vi "CRYO_MASTER_temp_0911.vi"() -> ()   [LabVIEW 2017] (continued)
s since 1904-01-01), timestamp(3682565793.190962 s since 1904-01-01), timestamp(3682565794.192923 s since 1904-01-01), timestamp(3682565795.1943216 s since 1904-01-01), timestamp(3682565796.1945167 s since 1904-01-01), timestamp(3682565797.194023 s since 1904-01-01), timestamp(3682565798.195678 s since 1904-01-01), timestamp(3682565799.194545 s since 1904-01-01), timestamp(3682565800.194017 s since 1904-01-01), timestamp(3682565801.196416 s since 1904-01-01), timestamp(3682565802.1962314 s since 1904-01-01), timestamp(3682565803.1960993 s since 1904-01-01), timestamp(3682565804.196091 s since 1904-01-01), timestamp(3682565805.197301 s since 1904-01-01)], "DataArray"=[99.5330106117578]}] caption="XY Graph"
  in  "log/linear 4":bool
  in  "log/linear 3":bool
  in  "float/scientific 1":bool
  in  "P_safelimit_up (Pa)":dbl=300000.0 format="%_4e"
  in  "P_safelimit_low (Pa)":dbl=100.0 format="%_4e"
  out "Pav - (P_2_th_high+P_2_tol)=":dbl
  in  "Auto ON?":bool
  out "Pstd history":dbl(graph)=554.7391446242465
  out "Pav history":dbl(graph)=-49199.19854911039
  in  "Mov. Avg Interval":i64=4
  in  "V2 (N.C.)":bool
  in  "V1 (N.O.)":bool=TRUE
  in  "N for sampling":i64=7
  in  "P_2_tol (Pa)":dbl=5000.0 format="%_4e"
  in  "P_1_tol (Pa)":dbl=5000.0 format="%_4e"
  in  "P_2_th_low (Pa)":dbl=1.03 format="%_4e"
  in  "P_1_th_low (Pa)":dbl=125000.0 format="%_4g"
  in  "P_2_th_high (Pa)":dbl=1.2 format="%_4e"
  in  "P_1_th_high (Pa)":dbl=130000.0 format="%_4e"
  out "Graph 5":T9(graph) caption="XY Graph"
  out "Last N M.A. Pressures":dbl[](array[numeric]) format="%_5e"
  out "Pav":dbl=-49199.19854911039 format="%0.4e"
  out "Pstd":dbl=554.7391446242465 format="%0.4e"
  out "Status V2 CTRL":enum16{"Pressurize", "Depressurize"}(ring)
  out "Status V1 CTRL":enum16{"Pressurize", "Depressurize"}(ring)
  out "Pav - (P_2_th_low_-P_2_tol)=":dbl
  out "Pav - (P_1_th_low_-P_1_tol)=":dbl
  out "Pav - (P_1_th_high+P_1_tol)=":dbl
  out "File Refn DewarCTRL":refnum<file>
  out "Error Out (Dewar CTRL":errorcluster
  out "Actual Current (mA)":dbl min=0.0 max=1.9
  out "Graph 7":T10(graph) caption="XY Graph"
  in  "upper limit (V)":dbl=20.0 format="%#_13g"
  in  "lower limit (V)":dbl format="%#_13g"
  in  "lower limit (mA)":dbl=4.0
  in  "upper limit (mA) 2":dbl=20.0
  in  "lower limit (mA)":dbl=4.0
  in  "SetCurrent 2 (mA)":dbl
  in  "upper limit (mA)":dbl=20.0
  out "error out (KIKUSI CTRL)":errorcluster={"status"=TRUE, "code"=1, "source"="Format Into String in FileWrite.vi->CRYO_MASTER_temp.vi"}
  out "ActualVoltage (V)":dbl[](array[numeric])
  out "ActualCurrent (A)":dbl[](array[numeric])=[0.008, 0.01]
  in  "SetCurrent 1 (mA)":dbl
  in  "Output":bool[](array[boolean])=[FALSE, FALSE]
  out "error out (ADCMT6420A)":errorcluster
  in  "Voltage limits (V)":dbl[](array[numeric])=[12.0, 12.0]
  in  "CtrlLabels":string[](array[string])=["CV2", "CV3"]
  in  "VISA":refnum<visa-resource-name>[](array[refnum])=["GPIB0::1::INSTR", "GPIB0::12::INSTR"]
  out "Initialized?":bool
  in  "InstName":string="ADCMT"
  out "Graph 6":T9(graph) caption="XY Graph"
  in  "Initialize":bool
  in  "CONTROL KIKUSUI?":bool=TRUE
  in  "OUTPUT":bool
  in  "Set Voltage (V)":dbl=20.0 min=0.0 max=49.0
  in  "Set Current (mA)":dbl=0.001 min=0.0 max=1.9
  in  "offset (mA)":dbl=10.0 format="%#_13g"
  out "Series 1":string[](array[string])=["P_Dewar"]
  out "Series 2":string[](array[string])=["T4He6", "T4He9", "T3He1-2", "T3He1-3", "T4He7", "T4He8", "T4He10", "T1K6", "TIP1", "N.C.", "TIP2", "T1K3-1", "T1K3-2", "T3He5", "T3He8", "T3He6-1", "T3He6-2", "T3He7-1", "T3He7-2"]
  out "Series 3":string[](array[string])=["P_ins", "P_4Kres", "P_3HeIN", "P_SldRTN", "P_3Hepot", "P_1Kepot", "DP_HEX4", "DP_HEX5"]
  out "Series 4":string[](array[string])=["L1", "L2-1", "L2-2", "L3"]
  out "Plot errors":errorcluster
  out "LastMeasurementConfig (218)":T11(array[cluster])=[{"LSIName"="LSI218A", "Active?"=TRUE, "LastData"=[297.63, 297.76, 296.71, 297.24, 295.38, 295.52, 294.91, 295.07], "Labels"=["T3He10", "T3He1-1", "TTH3", "TTH4", "TTH1", "TTH2", "T4He1", "T1K1"]}, {"LSIName"="LSI218B", "Active?"=TRUE, "LastData"=[30.0, 0.0, 0.0, 0.0, 296.58, 296.99, 295.68, 297.19], "Labels"=["N.C.", "N.C.", "N.C.", "N.C.", "T3He2-1", "T3He2-2", "T3He3", "T3He1-4"]}, {"LSIName"="LSI218C", "Active?"=TRUE, "LastData"=[297.39, 297.55, 297.28, 297.31, 296.61, 296.28, 296.32, 296.17], "Labels"=["T4He3-1", "T4He3-2", "T4He3-3", "T4He3-4", "T4He2-1", "T4He2-2", "T4He4", "T4He5"]}, {"LSIName"="LSI218D", "Active?"=TRUE, "LastData"=[296.4, 297.17, 297.92, 297.51, 296.71, 297.02, 296.96, 297.42], "Labels"=["T4He6", "T4He9", "T3He1-2", "T3He1-3", "T4He7", "T4He8", "T4He10", "T1K6"]}, {"LSIName"="LSI218E", "Active?"=TRUE, "LastData"=[296.77, 0.0, 296.31, 688.49, 296.06, 295.63, 295.73, 688.58], "Labels"=["TIP1", "N.C.", "TIP2", "N.C.", "TIP3", "TIP4", "TIP5", "N.C."]}, {"LSIName"="LSI218F", "Active?"=TRUE, "LastData"=[302.11, 301.08, 296.91, 291.77, 288.69, 280.14, 0.433, 0.0], "Labels"=["T1K2", "T1K4", "T1K5", "T3He4", "T3He9", "TIP6", "N.C.", "N.C."]}]
  out "DataArrayConv (USB6210)":dbl[][](array[numeric])=[[0.000981756523507472, 101282.93029464335, 100447.56177003749, 100215.69769894995, 100421.61018172985, 100780.20754019849, 98878.77979362432, -9.626849444535207, 78.6252889928285, 100.08609659349952, 0.1296859810079549, 0.1356046075893618, 99.5330106117578]]
  out "LastMeasurementConfig (336)":T11(array[cluster])=[{"LSIName"="LSi336X", "Active?"=TRUE, "LastData"=[296.838, 296.434, 296.022, 296.217], "Labels"=["T1K3-1", "T1K3-2", "T3He5", "T3He8"]}, {"LSIName"="LSi336Y", "Active?"=TRUE, "LastData"=[295.887, 295.842, 295.916, 296.504], "Labels"=["T3He6-1", "T3He6-2", "T3He7-1", "T3He7-2"]}]
  out "DataArrayConv (USB6218)":dbl[][](array[numeric])
  out "TimeArray (USB6218)":timestamp[](array[timestamp])
  # "GLOBAL STATUS/CONTROL"
  # "USB6210 Analog inputs Settings"
  # "USB6218 Analog inputs Settings"
  # "USB6218 Digital Output Settings"
  # "USB6218 Analog Output Settings"
  # "Global Settings"
  # "LSI218 Settings"
  # "LSI336 Settings"
  # "Graph screenshots"
  # "Configuration"
  # "Vavle Status"
  # "OPEN"
  # "CLOSED"
  # "ADCMT6240A Control/Status"
  # "ADCMT6240A Initialization"
  # "Set Currents (mA)"
  # "KIKUSUI PWR400H CTRL via USB6218"
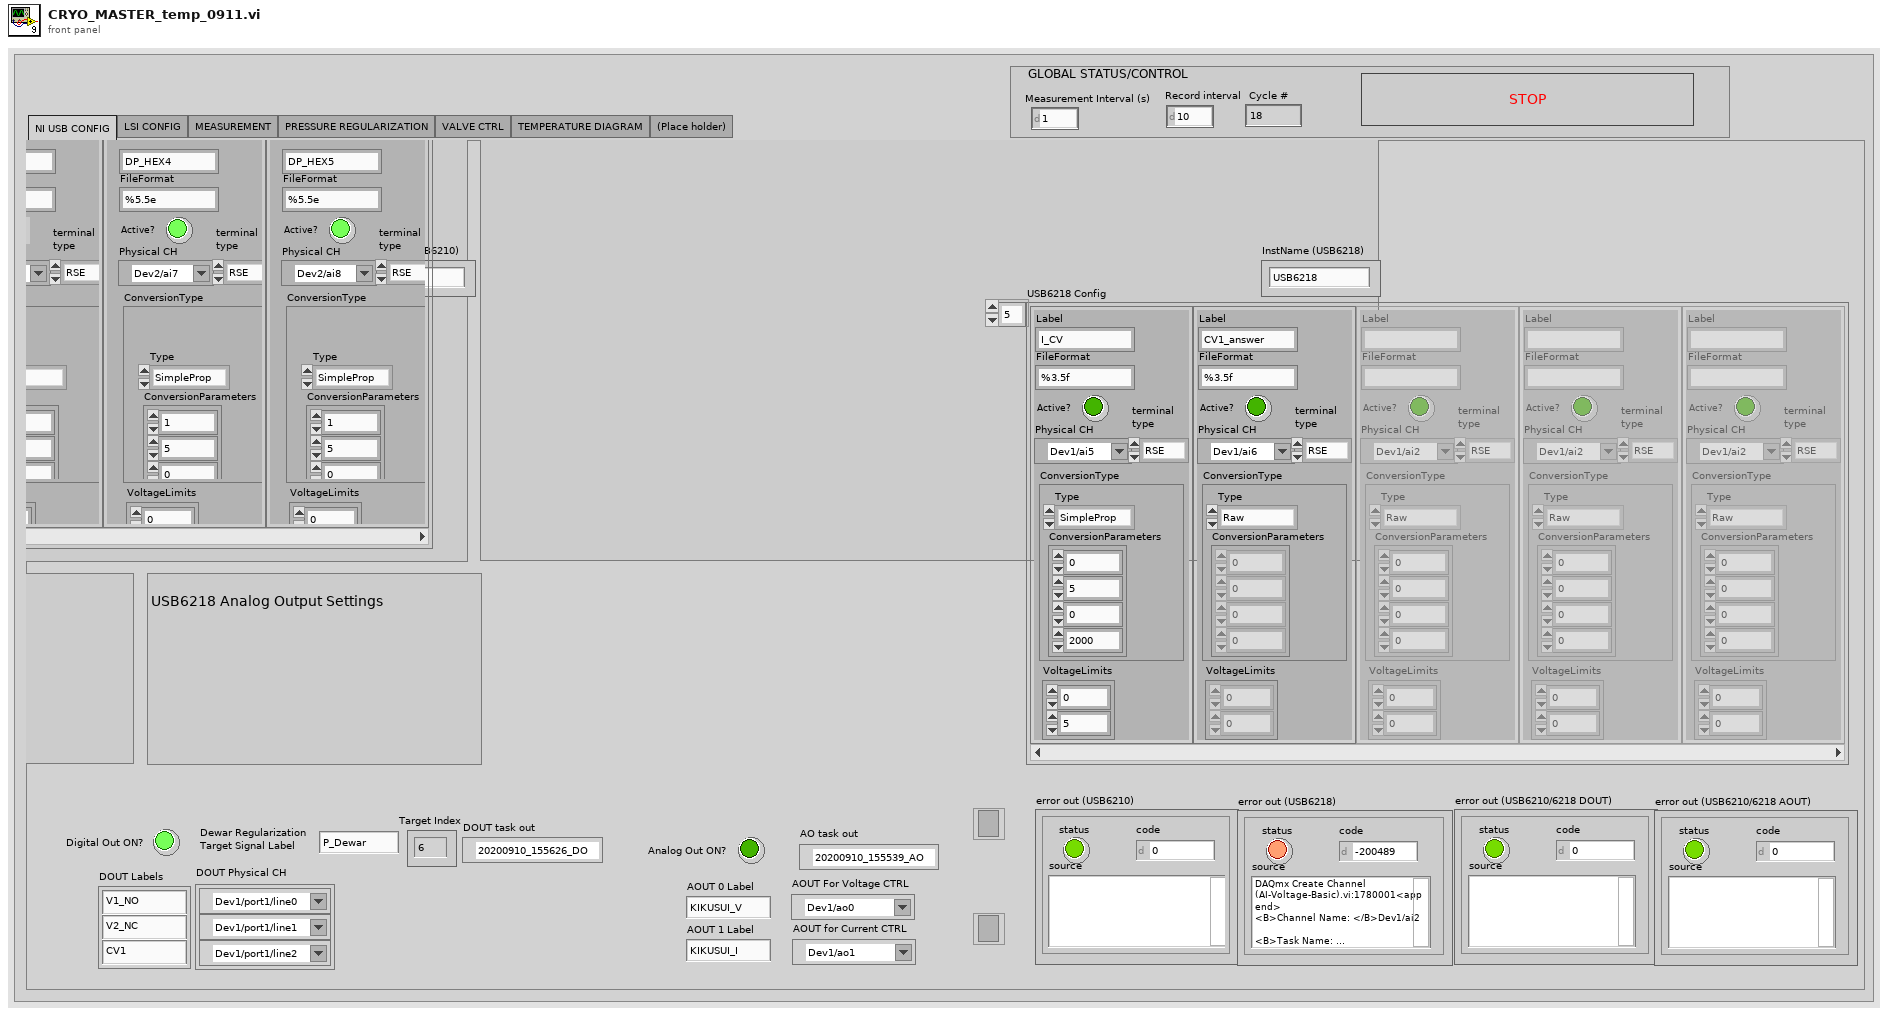
[diagram p1: front panel]
types:
  T1 = enum32{"NI USB CONFIG", "LSI CONFIG", "MEASUREMENT", "PRESSURE REGULARIZATION", "VALVE CTRL", "TEMPERATURE DIAGRAM", "(Place holder)"}
  T2 = cluster{"Label":string, "FileFormat":string, "Active?":bool, "Physical CH":tag, " terminal\n type":i32, "ConversionType":cluster{"Type":enum16{"Raw", "SimpleProp", "CC-10_COMBINED", "CC-10_LOG", "LeakDet_EXP", "LeakDet_Mantissa", "Baratron"}, "ConversionParameters":dbl[]}, "VoltageLimits":dbl[]}[]
  T3 = cluster{"LSIName":string, "Labels":string[], "SensorLocations":enum16{"N.C.", "T3He1-1", "T3He1-2", "T3He1-3", "T3He1-4", "T3He2-1", "T3He2-2", "T3He3", "T3He4", "T3He5", "T3He6-1", "T3He6-2", "T3He7-1", "T3He7-2", "T3He8", "T3He9", "T3He10", "T4He1", "T4He2-1", "T4He2-2", "T4He3-1", "T4He3-2", "T4He3-3", "T4He3-4", "T4He4", "T4He5", "T4He6", "T4He7", "T4He8", "T4He9", "T4He10", "T1K1", "T1K2", "T1K3-1", "T1K3-2", "T1K4", "T1K5", "T1K6", "TIP1", "TIP2", "TIP3", "TIP4", "TIP5", "TIP6", "TIP7", "TTH1", "TTH2", "TTH3", "TTH4"}[], "Active?":bool, "VISA res. name":refnum<visa-resource-name>}[]
  T4 = enum32{"USB6210", "USB6218", "Temeprature (1)", "Temperature (2)", "Temperature (3)"}
  T5 = enum16{"Intialized", "Ready", "Measuring", "Terminated"}
  T6 = enum16{"Initialized", "Ready", "Measuring", "Terminated"}
  T7 = cluster{"TimeArray":timestamp[], "LDArray":dbl[]}[]
  T8 = cluster{"TimeArray":timestamp[], "DataArray":dbl[]}[]
  T9 = cluster{"TimeArray":timestamp[], "Filtered X":dbl[]}[]
  T10 = cluster{"TimeArray (USB6218)":timestamp[], "DataArrayConv (USB6218)":dbl[]}[]
  T11 = cluster{"LSIName":string, "Active?":bool, "LastData":dbl[], "Labels":string[]}[]
  T12 = cluster{"TimeArray (USB6218)":timestamp[], "DataArrayConv (USB6218)":dbl[]}
  T13 = enum16{"open", "replace", "create", "open or create", "replace or create", "replace or create with confirmation"}
  T14 = cluster{"TimeArray":timestamp[], "DataArrayConv":dbl[]}[]
  T15 = cluster{"IndexArray":i64[], "TimeArray":timestamp[], "DataArrayRaw":dbl[][], "DataArrayConv":dbl[][], "LDArray":dbl[]}
  T16 = cluster{"InstName":string, "Active?":bool, "Status":enum16{"Intialized", "Ready", "Measuring", "Terminated"}, "Labels":string[], "LabelLD":string, "FileFormat":string[], "FileFormatLD":string, "ReadLeakDet?":bool}
  T17 = cluster{"TimeArray":timestamp[], "DataArrayConv":dbl[]}
  T18 = cluster{"TimeArray":timestamp[], "DataArray":dbl[]}
  T19 = cluster{"TimeArray":timestamp[], "Filtered X":dbl[]}
  T20 = cluster{"appended array":timestamp[], "ActualCurrentArray":dbl[]}
  T21 = cluster{"appended array":timestamp[], "SetCurrentArray":dbl[]}
  T22 = cluster{"appended array":timestamp[], "SetCurrentArray":dbl[]}[]
diagram:
  w3 = errorcluster {"status"=FALSE, "code"=0, "source"=""} ("error in (no error)")
  n1 = while {
    shift-right: [w38] -> _
    shift-left: dbl[] [] -> [w43]
    shift-right: [w39] -> _
    shift-left: timestamp[] [] -> [w42]
    i -> [w41]
    stop <- w51 stop-if-true
    n2 = stacked-sequence {
      tunnel: "upper limit (V)" -> [w58 w66 _]
      tunnel: "upper limit (mA) 2" -> [w56 w64 _]
      tunnel: "lower limit (V)" -> [w54 w62 _]
      tunnel: "Set Current (mA)" -> [w53 _ _]
      tunnel: [_ _ w73] -> w46
      tunnel: "Set Voltage (V)" -> [_ w61 _]
      tunnel: [_ _ w72] -> w44
      frame #0 {
        n3 = Greater?(x=w53, y=w58) -> (0:w57:bool)
        n4 = Less?(x=w53, y=w54) -> (x < y?=w55:bool)
        n5 = case shown="True" w57 {
          tunnel: w56 -> [_ w60]
          frame False {
          }
          frame True {
            n6 = property on="Set Current (mA)" class="DigNum (strict)"("Val(Sgnl)"=w60) -> ()  [unwired: 2 in, 2 out]
          }
        }
        n7 = case shown="True" w55 {
          tunnel: w54 -> [_ w59]
          frame False {
          }
          frame True {
            n8 = property on="Set Current (mA)" class="DigNum (strict)"("Val(Sgnl)"=w59) -> ()  [unwired: 2 in, 2 out]
          }
        }
      }
      frame #1 {
        n9 = Greater?(x=w61, y=w66) -> (0:w65:bool)
        n10 = Less?(x=w61, y=w62) -> (x < y?=w63:bool)
        n11 = case shown="True" w65 {
          tunnel: w64 -> [_ w68]
          frame False {
          }
          frame True {
            n12 = property on="Set Voltage (V)" class="DigNum (strict)"("Val(Sgnl)"=w68) -> ()  [unwired: 2 in, 2 out]
          }
        }
        n13 = case shown="True" w63 {
          tunnel: w62 -> [_ w67]
          frame False {
          }
          frame True {
            n14 = property on="Set Voltage (V)" class="DigNum (strict)"("Val(Sgnl)"=w67) -> ()  [unwired: 2 in, 2 out]
          }
        }
      }
      frame #2 {
        n15 = property on="Set Current (mA)" class="DigNum (strict)"() -> ("Value"=w71:dbl)  [unwired: 2 in, 2 out]
        n16 = Add(x=w71, y="offset (mA)") -> (x+y=w69:dbl)
        n17 = property on="Set Voltage (V)" class="DigNum (strict)"() -> ("Value"=w72:dbl)  [unwired: 2 in, 2 out]
        n18 = Divide(x=w69, y=1000.0) -> (x/y=w73:dbl)
      }
    }
    n19 = Wait (ms)(milliseconds to wait=u32 25) -> ()  [unwired: 1 out]
    n20 = event shown="[4] \"CONTROL KIKUSUI?\", \"Set Voltage (V)\", \"Set Current (mA)\": Value Change" {
      selector: _ -> [_ _ _ _ _ _]
      dyn-events: _ -> [_ _ _ _ _ _]
      timeout: _ -> [_ _ _ _ _ _]
      tunnel: [_ TRUE _ _ _ _] -> w51
      tunnel: w46 -> [_ _ _ _ w136 _]
      tunnel: w44 -> [_ _ _ _ w135 _]
      tunnel: w41 -> [_ _ _ _ w134 _]
      tunnel: [w76 w78 _ _ w133 w179] -> w38
      tunnel: w43 -> [w76 w78 _ _ w130 w179]
      tunnel: [w75 w77 _ _ w132 w180] -> w39
      tunnel: w42 -> [w75 w77 _ _ w131 w180]
      tunnel: w41 -> [_ _ w86 w107 _ w181]
      event Timeout {
        n21 = event-data() -> ()  [unwired: 1 in, 3 out]
      }
      event "Stop Button": Value Change {
        n22 = event-data() -> ()  [unwired: 1 in, 3 out]
        n23 = local read "AO task out"() -> (w80:refnum<k21>)
        n24 = local read "DOUT task out"() -> (w83:refnum<k21>)
        n25 = call <vilib>:"DAQmx Clear Task.vi"("task in"=w80, "error in"=errorcluster {"status"=FALSE, "code"=0, "source"=""}) -> ("error out"=w79:errorcluster)  [unwired: 13 in]
        n26 = call <vilib>:"DAQmx Clear Task.vi"("task in"=w83, "error in"=errorcluster {"status"=FALSE, "code"=0, "source"=""}) -> ("error out"=w84:errorcluster)  [unwired: 13 in]
        n27 = local write "error out (USB6210/6218 AOUT)"(w79) -> ()
        n28 = local write "error out (USB6210/6218 DOUT)"(w84) -> ()
      }
      event "V1 (N.O.)": Value Change {
        n29 = event-data() -> ()  [unwired: 1 in, 3 out]
        n30 = local read "Cycle #"() -> (w89:u32)
        n31 = Greater?(x=w89, y=u32 0) -> (0:w87:bool)
        n32 = case shown="True" w87 {
          tunnel: "V1 (N.O.)" -> [_ w99]
          tunnel: w86 -> [_ w94]
          frame False {
          }
          frame True {
            n33 = Not(x=w99) -> (.not. x?=w103:bool)
            n34 = local read "File Refn USB DO"() -> (w95:refnum<file>)
            n35 = local read "error out (USB6210/6218 DOUT)"() -> (w101:errorcluster)
            n36 = Initialize Array("%d" ("element"), 3 ("dimension size")) -> (w93:string[])
            n37 = property on="V2 (N.C.)" class="Bool (strict)"() -> ("Value"=w98:bool)  [unwired: 2 in, 2 out]
            n38 = property on="OUTPUT" class="Bool (strict)"() -> ("Value"=w97:bool)  [unwired: 2 in, 2 out]
            n39 = local read "DOUT task out"() -> (w106:refnum<k21>)
            n40 = Get Date/Time In Seconds() -> (seconds since 1Jan1904=w96:timestamp)
            n41 = call "FileWrite.vi"("Time Stamp"=w96, "FileFormat"=w93, "Index"=w94, "refnum in"=w95) -> ()  [unwired: 6 in, 2 out]
            n42 = Build Array(w103, w98, w97) -> (w102:bool[])
            n43 = call <vilib>:"DAQmx Write (Digital 1D Bool NChan 1Samp 1Line).vi"("task/channels in"=w106, "data"=w102, "timeout"=10.0, "error in"=w101) -> ("task out"=w104:refnum<k21>, "error out"=w100:errorcluster)  [unwired: 9 in, 1 out]
            n44 = local write "DOUT task out"(w104) -> ()
            n45 = local write "error out (USB6210/6218 DOUT)"(w100) -> ()
          }
        }
      }
      event "V2 (N.C.)": Value Change {
        n46 = event-data() -> ()  [unwired: 1 in, 3 out]
        n47 = local read "Cycle #"() -> (w110:u32)
        n48 = Greater?(x=w110, y=u32 0) -> (0:w108:bool)
        n49 = case shown="True" w108 {
          tunnel: "V2 (N.C.)" -> [_ w125]
          tunnel: w107 -> [_ w117]
          frame False {
          }
          frame True {
            n50 = property on="V1 (N.O.)" class="Bool (strict)"() -> ("Value"=w124:bool)  [unwired: 2 in, 2 out]
            n51 = local read "error out (USB6210/6218 DOUT)"() -> (w128:errorcluster)
            n52 = Not(x=w124) -> (.not. x?=w123:bool)
            n53 = property on="OUTPUT" class="Bool (strict)"() -> ("Value"=w122:bool)  [unwired: 2 in, 2 out]
            n54 = local read "DOUT task out"() -> (w129:refnum<k21>)
            n55 = Build Array(w123, w125, w122) -> (w120:bool[])
            n56 = local read "File Refn USB DO"() -> (w121:refnum<file>)
            n57 = Boolean To (0,1)(Boolean=w120) -> (0, 1=w119:i16[])
            n58 = call <vilib>:"DAQmx Write (Digital 1D Bool NChan 1Samp 1Line).vi"("task/channels in"=w129, "data"=w120, "timeout"=10.0, "error in"=w128) -> ("task out"=w126:refnum<k21>, "error out"=w113:errorcluster)  [unwired: 9 in, 1 out]
            n59 = Initialize Array("%d" ("element"), 3 ("dimension size")) -> (w114:string[])
            n60 = Get Date/Time In Seconds() -> (seconds since 1Jan1904=w118:timestamp)
            n61 = local write "DOUT task out"(w126) -> ()
            n62 = call "FileWrite.vi"("DataArray"=w119, "Time Stamp"=w118, "Error In"=w113, "FileFormat"=w114, "Index"=w117, "refnum in"=w121) -> ("Error Out"=w112:errorcluster)  [unwired: 4 in, 1 out]
            n63 = local write "error out (USB6210/6218 DOUT)"(w112) -> ()
          }
        }
      }
      event "CONTROL KIKUSUI?", "Set Voltage (V)", "Set Current (mA)": Value Change {
        n64 = event-data() -> ()  [unwired: 1 in, 3 out]
        n65 = case shown="True" "CONTROL KIKUSUI?" {
          tunnel: w136 -> [_ w153]
          tunnel: w135 -> [_ w158]
          tunnel: w134 -> [_ w161]
          tunnel: [w138 w151] -> w133
          tunnel: [w141 w150] -> w132
          tunnel: w131 -> [w143 w154]
          tunnel: w130 -> [w139 w152]
          frame False {
            w140 = 0.0 ("element")
            n66 = Get Date/Time In Seconds() -> (seconds since 1Jan1904=w142:timestamp)
            n67 = local read "AO task out"() -> (w148:refnum<k21>)
            n68 = Build Array (concatenate)(w143, w142) -> (w141:timestamp[])
            n69 = Build Array (concatenate)(w139, w140) -> (w138:dbl[])
            n70 = Build Array(w140, w140) -> (w146:dbl[])
            n71 = call <vilib>:"DAQmx Write (Analog 1D DBL NChan 1Samp).vi"("task/channels in"=w148, "data"=w146, "timeout"=100.0, "error in"=errorcluster {"status"=FALSE, "code"=0, "source"=""}) -> ("task out"=w149:refnum<k21>, "error out"=w144:errorcluster)  [unwired: 9 in, 1 out]
            n72 = local write "AO task out"(w149) -> ()
            n73 = local write "error out (KIKUSI CTRL)"(w144) -> ()
          }
          frame True {
            n74 = Build Array(w158, w153) -> (w156:dbl[])
            n75 = Divide(x=w153, y=2.0) -> (x/y=w171:dbl)
            n76 = Divide(x=w158, y=650.0) -> (x/y=w174:dbl)
            n77 = local read "File Refn USB AO"() -> (w162:refnum<file>)
            n78 = Multiply(x=10.0 ("y"), y=w174) -> (x*y=w169:dbl)
            n79 = Multiply(x=w171, y=10.0) -> (x*y=w168:dbl)
            n80 = Build Array(w169, w168) -> (w167:dbl[])
            n81 = Initialize Array("%.3f", 2 ("dimension size")) -> (w163:string[])
            n82 = Get Date/Time In Seconds() -> (seconds since 1Jan1904=w155:timestamp)
            n83 = local read "AO task out"() -> (w176:refnum<k21>)
            n84 = call "FileWrite.vi"("DataArray"=w156, "Time Stamp"=w155, "Error In"=errorcluster {"status"=FALSE, "code"=0, "source"=""} ("error in"), "FileFormat"=w163, "Index"=w161, "refnum in"=w162) -> ("Error Out"=w159:errorcluster, "Byte Stream File Refnum"=w157:refnum<file>)  [unwired: 4 in]
            n85 = Build Array (concatenate)(w154, w155) -> (w150:timestamp[])
            n86 = Build Array (concatenate)(w152, w153) -> (w151:dbl[])
            n87 = local write "File Refn USB AO"(w157) -> ()
            n88 = call <vilib>:"DAQmx Write (Analog 1D DBL NChan 1Samp).vi"("task/channels in"=w176, "data"=w167, "timeout"=100.0, "error in"=w159) -> ("task out"=w177:refnum<k21>, "error out"=→"error out (KIKUSI CTRL)":errorcluster)  [unwired: 9 in, 1 out]
            n89 = local write "AO task out"(w177) -> ()
          }
        }
      }
      event "OUTPUT": Value Change {
        n90 = event-data() -> ()  [unwired: 1 in, 6 out]
        n91 = local read "Cycle #"() -> (w184:u32)
        n92 = Greater?(x=w184, y=u32 0) -> (0:w182:bool)
        n93 = case shown="True" w182 {
          tunnel: w181 -> [_ w188]
          frame False {
          }
          frame True {
            n94 = property on="V1 (N.O.)" class="Bool (strict)"() -> ("Value"=w199:bool)  [unwired: 2 in, 2 out]
            n95 = local read "error out (USB6210/6218 DOUT)"() -> (w202:errorcluster)
            n96 = Not(x=w199) -> (.not. x?=w198:bool)
            n97 = property on="V2 (N.C.)" class="Bool (strict)"() -> ("Value"=w197:bool)  [unwired: 2 in, 2 out]
            n98 = local read "DOUT task out"() -> (w203:refnum<k21>)
            n99 = Build Array(w198, w197, "OUTPUT") -> (w186:bool[])
            n100 = Boolean To (0,1)(Boolean=w186) -> (0, 1=w185:i16[])
            n101 = local read "File Refn USB DO"() -> (w189:refnum<file>)
            n102 = call <vilib>:"DAQmx Write (Digital 1D Bool NChan 1Samp 1Line).vi"("task/channels in"=w203, "data"=w186, "timeout"=10.0, "error in"=w202) -> ("task out"=w200:refnum<k21>, "error out"=w193:errorcluster)  [unwired: 9 in, 1 out]
            n103 = Initialize Array("%d" ("element"), 3 ("dimension size")) -> (w191:string[])
            n104 = local write "DOUT task out"(w200) -> ()
            n105 = Get Date/Time In Seconds() -> (seconds since 1Jan1904=w190:timestamp)
            n106 = call "FileWrite.vi"("DataArray"=w185, "Time Stamp"=w190, "Error In"=w193, "FileFormat"=w191, "Index"=w188, "refnum in"=w189) -> ("Error Out"=w192:errorcluster, "Byte Stream File Refnum"=w187:refnum<file>)  [unwired: 4 in]
            n107 = local write "File Refn USB DO"(w187) -> ()
            n108 = local write "error out (USB6210/6218 DOUT)"(w192) -> ()
          }
        }
      }
    }
    n109 = local read "All Labels (USB6218)"() -> (w30:string[])
    n110 = Search 1D Array(1D array=w30, element="I_CV") -> (index of element=w28:i32)  [unwired: 1 in]
    n111 = local read "Last Data \n(USB6218)"() -> (w35:dbl[])
    n112 = Index Array(array=w35, index=w28) -> (element=→"Actual Current (mA)":dbl)
    n113 = local read "DataArrayConv (USB6218)"() -> (w31:dbl[][])
    n114 = Index Array(array=w31, index (row)=w28) -> (element=w32:dbl[])  [unwired: 1 in]
    n115 = local read "TimeArray (USB6218)"() -> (w33:timestamp[])
    n116 = Bundle(w39, w38) -> (w37:cluster{timestamp[], dbl[]})  [unwired: 1 in]
    n117 = Bundle("TimeArray (USB6218)"=w33, "DataArrayConv (USB6218)"=w32) -> (w36:T12)  [unwired: 1 in]
    n118 = Build Array(w37, w36) -> (→"Graph 7":T10)
  }
  n119 = while {
    stop <- w207 stop-if-true
    n120 = event shown="[5] \"float/scientific 1\": Value Change" {
      selector: _ -> [_ _ _ _ _ _ _ _ _ _ _ _]
      dyn-events: _ -> [_ _ _ _ _ _ _ _ _ _ _ _]
      timeout: _ -> [_ _ _ _ _ _ _ _ _ _ _ _]
      tunnel: [_ _ _ _ _ _ _ _ _ _ _ TRUE] -> w207
      event Timeout {
        n121 = event-data() -> ()  [unwired: 1 in, 3 out]
      }
      event "log/linear 1": Value Change {
        n122 = event-data() -> ()  [unwired: 1 in, 6 out]
        n123 = flat-sequence {
          frame #0 {
            n124 = control-ref of="Graph 1"() -> (w213:refnum<vi>)
            n125 = Boolean To (0,1)(Boolean="log/linear 1") -> (0, 1=w214:i16)
            n126 = property class="XYGraph (strict)"(reference=w213, error in=errorcluster {"status"=FALSE, "code"=0, "source"=""} ("error in (no error)"), "YScale.Mapping Mode"=w214) -> (error out=w211:errorcluster)  [unwired: 1 out]
            n127 = control-ref of="error out (USB6210)"() -> (w212:refnum<vi>)
            n128 = property class="Clust (strict)"(reference=w212, "Val(Sgnl)"=w211) -> ()  [unwired: 1 in, 2 out]
          }
        }
      }
      event "log/linear 2": Value Change {
        n129 = event-data() -> ()  [unwired: 1 in, 6 out]
        n130 = flat-sequence {
          frame #0 {
            n131 = control-ref of="Graph 2"() -> (w218:refnum<vi>)
            n132 = Boolean To (0,1)(Boolean="log/linear 2") -> (0, 1=w220:i16)
            n133 = property class="XYGraph (strict)"(reference=w218, error in=errorcluster {"status"=FALSE, "code"=0, "source"=""} ("error in (no error)"), "YScale.Mapping Mode"=w220) -> (error out=w219:errorcluster)  [unwired: 1 out]
            n134 = control-ref of="error out (USB6210)"() -> (w217:refnum<vi>)
            n135 = property class="Clust (strict)"(reference=w217, "Value"=w219) -> ()  [unwired: 1 in, 2 out]
          }
        }
      }
      event "log/linear 3": Value Change {
        n136 = event-data() -> ()  [unwired: 1 in, 6 out]
        n137 = flat-sequence {
          frame #0 {
            n138 = control-ref of="Graph 3"() -> (w222:refnum<vi>)
            n139 = Boolean To (0,1)(Boolean="log/linear 3") -> (0, 1=w226:i16)
            n140 = property class="XYGraph (strict)"(reference=w222, error in=errorcluster {"status"=FALSE, "code"=0, "source"=""} ("error in (no error)"), "YScale.Mapping Mode"=w226) -> (error out=w225:errorcluster)  [unwired: 1 out]
            n141 = control-ref of="error out (USB6210)"() -> (w224:refnum<vi>)
            n142 = property class="Clust (strict)"(reference=w224, "Value"=w225) -> ()  [unwired: 1 in, 2 out]
          }
        }
      }
      event "log/linear 4": Value Change {
        n143 = event-data() -> ()  [unwired: 1 in, 6 out]
        n144 = flat-sequence {
          frame #0 {
            n145 = control-ref of="Graph 4"() -> (w228:refnum<vi>)
            n146 = Boolean To (0,1)(Boolean="log/linear 4") -> (0, 1=w232:i16)
            n147 = property class="XYGraph (strict)"(reference=w228, error in=errorcluster {"status"=FALSE, "code"=0, "source"=""} ("error in (no error)"), "YScale.Mapping Mode"=w232) -> (error out=w231:errorcluster)  [unwired: 1 out]
            n148 = control-ref of="error out (USB6210)"() -> (w230:refnum<vi>)
            n149 = property class="Clust (strict)"(reference=w230, "Value"=w231) -> ()  [unwired: 1 in, 2 out]
          }
        }
      }
      event "float/scientific 1": Value Change {
        n150 = event-data() -> ()  [unwired: 1 in, 6 out]
        n151 = flat-sequence {
          frame #0 {
            n152 = control-ref of="Graph 4"() -> (w236:refnum<vi>)
            n153 = case shown="False" "float/scientific 1" {
              tunnel: [u8 1 ("Y Scale.Display Format:Format") u8 2 ("Y Scale.Display Format:Format")] -> w235
              frame False {
              }
              frame True {
              }
            }
            n154 = property class="XYGraph (strict)"(reference=w236, error in=errorcluster {"status"=FALSE, "code"=0, "source"=""} ("error in (no error)"), "YScale.Format"=w235) -> (error out=w238:errorcluster)  [unwired: 1 out]
            n155 = control-ref of="error out (USB6210)"() -> (w237:refnum<vi>)
            n156 = property class="Clust (strict)"(reference=w237, "Value"=w238) -> ()  [unwired: 1 in, 2 out]
          }
        }
      }
      event "Plot selecter LSI218(1)\n    1      2     3     4", "Plot selecter LSI218(2)\n    1      2     3     4", "Plot selecter (USB6210)\n    1      2     3     4", "Plot selecter LSI336 \n     1      2     3     4", "Plot selecter (USB6218)\n    1      2     3     4": Value Change {
        n157 = event-data() -> ()  [unwired: 1 in, 6 out]
        n158 = local read "All Labels (USB6210)"() -> (w258:string[])
        n159 = local read "All Labels (USB6218)"() -> (w247:string[])
        n160 = local read "Labels LSI218 (1)"() -> (w260:string[])
        n161 = local read "Labels LSI218 (2)"() -> (w261:string[])
        n162 = local read "Labels LSI336"() -> (w253:string[])
        n163 = call "BuildPlotLegends.vi"("Plot selecter \n    1      2     3     4"="Plot selecter (USB6210)\n    1      2     3     4", "AllLabels"=w258) -> ("Series 4"=w270:string[], "Series 3"=w268:string[], "Series 2"=w266:string[], "Series 1"=w264:string[])  [unwired: 6 in]
        n164 = call "BuildPlotLegends_LSI218.vi"("Plot selecter (2)\n    1      2     3     5"="Plot selecter LSI218(2)\n    1      2     3     4", "Plot selecter (1)\n    1      2     3     4"="Plot selecter LSI218(1)\n    1      2     3     4", "Labels (2)"=w261, "Labels (1)"=w260) -> ("Series 4"=w271:string[], "Series 3"=w269:string[], "Series 2"=w267:string[], "Series 1"=w265:string[])  [unwired: 4 in]
        n165 = call "BuildPlotLegends.vi"("Plot selecter \n    1      2     3     4"="Plot selecter LSI336 \n     1      2     3     4", "AllLabels"=w253) -> ("Series 4"=w248:string[], "Series 3"=w249:string[], "Series 2"=w250:string[], "Series 1"=w251:string[])  [unwired: 6 in]
        n166 = call "BuildPlotLegends.vi"("Plot selecter \n    1      2     3     4"="Plot selecter (USB6218)\n    1      2     3     4", "AllLabels"=w247) -> ("Series 4"=w243:string[], "Series 3"=w242:string[], "Series 2"=w244:string[], "Series 1"=w245:string[])  [unwired: 6 in]
        n167 = Build Array (concatenate)(w266, w267, w250, w244) -> (w255:string[])
        "Series 2" <- w255
        n168 = Build Array (concatenate)(w268, w269, w249, w242) -> (w256:string[])
        "Series 3" <- w256
        n169 = Build Array (concatenate)(w270, w271, w248, w243) -> (w257:string[])
        "Series 4" <- w257
        n170 = Build Array (concatenate)(w264, w265, w251, w245) -> (w254:string[])
        "Series 1" <- w254
        n171 = stacked-sequence {
          tunnel: [w280 _ _ _] -> w275
          tunnel: [_ w299 _ _] -> w276
          tunnel: [_ _ w315 _] -> w274
          tunnel: [_ _ _ w332] -> w273
          tunnel: w254 -> [w277 _ _ _]
          tunnel: w255 -> [_ w295 _ _]
          tunnel: w256 -> [_ _ w312 _]
          tunnel: w257 -> [_ _ _ w329]
          frame #0 {
            n172 = Array Size(array=w277) -> (size(s)=w283:i32)
            n173 = control-ref of="Graph 1"() -> (w281:refnum<vi>)
            n174 = for {
              N: 18 -> [_]
              tunnel: w281 -> [w292]
              shift-right: [w290] -> w282
              shift-left: errorcluster {"status"=FALSE, "code"=0, "source"=""} ("error in (no error)") -> [w291]
              i -> [w294]
              n175 = property class="XYGraph (strict)"(reference=w292, error in=w291, "Active Plot"=w294, "Plot.Plot Name"="") -> (error out=w290:errorcluster)  [unwired: 1 out]
            }
            n176 = for {
              N: w283 -> [_]
              tunnel: w281 -> [w288]
              shift-right: [w286] -> w280
              shift-left: w282 -> [w287]
              tunnel: w277 -> [w285] mode=indexing
              i -> [w289]
              n177 = property class="XYGraph (strict)"(reference=w288, error in=w287, "Active Plot"=w289, "Plot.Plot Name"=w285, "Plot.Visible?"=TRUE ("Plot.Visible")) -> (error out=w286:errorcluster)  [unwired: 1 out]
            }
          }
          frame #1 {
            n178 = Array Size(array=w295) -> (size(s)=w301:i32)
            n179 = control-ref of="Graph 2"() -> (w298:refnum<vi>)
            n180 = for {
              N: 18 -> [_]
              shift-right: [w308] -> w300
              shift-left: errorcluster {"status"=FALSE, "code"=0, "source"=""} ("error in (no error)") -> [w309]
              tunnel: w298 -> [w307]
              i -> [w311]
              n181 = property class="XYGraph (strict)"(reference=w307, error in=w309, "Active Plot"=w311, "Plot.Plot Name"="") -> (error out=w308:errorcluster)  [unwired: 1 out]
            }
            n182 = for {
              N: w301 -> [_]
              shift-right: [w304] -> w299
              shift-left: w300 -> [w305]
              tunnel: w295 -> [w303] mode=indexing
              tunnel: w298 -> [w302]
              i -> [w306]
              n183 = property class="XYGraph (strict)"(reference=w302, error in=w305, "Active Plot"=w306, "Plot.Plot Name"=w303) -> (error out=w304:errorcluster)  [unwired: 1 out]
            }
          }
          frame #2 {
            n184 = Array Size(array=w312) -> (size(s)=w318:i32)
            n185 = control-ref of="Graph 3"() -> (w316:refnum<vi>)
            n186 = for {
              N: 18 -> [_]
              tunnel: w316 -> [w326]
              shift-right: [w324] -> w317
              shift-left: errorcluster {"status"=FALSE, "code"=0, "source"=""} ("error in (no error)") -> [w325]
              i -> [w328]
              n187 = property class="XYGraph (strict)"(reference=w326, error in=w325, "Active Plot"=w328, "Plot.Plot Name"="") -> (error out=w324:errorcluster)  [unwired: 1 out]
            }
            n188 = for {
              N: w318 -> [_]
              tunnel: w316 -> [w322]
              shift-right: [w320] -> w315
              shift-left: w317 -> [w321]
              tunnel: w312 -> [w319] mode=indexing
              i -> [w323]
              n189 = property class="XYGraph (strict)"(reference=w322, error in=w321, "Active Plot"=w323, "Plot.Plot Name"=w319) -> (error out=w320:errorcluster)  [unwired: 1 out]
            }
          }
          frame #3 {
            n190 = Array Size(array=w329) -> (size(s)=w335:i32)
            n191 = control-ref of="Graph 4"() -> (w333:refnum<vi>)
            n192 = for {
              N: 18 -> [_]
              tunnel: w333 -> [w343]
              shift-right: [w341] -> w334
              shift-left: errorcluster {"status"=FALSE, "code"=0, "source"=""} ("error in (no error)") -> [w342]
              i -> [w345]
              n193 = property class="XYGraph (strict)"(reference=w343, error in=w342, "Active Plot"=w345, "Plot.Plot Name"="") -> (error out=w341:errorcluster)  [unwired: 1 out]
            }
            n194 = for {
              N: w335 -> [_]
              tunnel: w333 -> [w339]
              shift-right: [w337] -> w332
              shift-left: w334 -> [w338]
              tunnel: w329 -> [w336] mode=indexing
              i -> [w340]
              n195 = property class="XYGraph (strict)"(reference=w339, error in=w338, "Active Plot"=w340, "Plot.Plot Name"=w336) -> (error out=w337:errorcluster)  [unwired: 1 out]
            }
          }
        }
        n196 = Merge Errors(w275, w276, w274, w273) -> (→"Plot errors":errorcluster)
      }
      event "Take Screenshot! 1": Value Change {
        n197 = event-data() -> ()  [unwired: 1 in, 6 out]
        n198 = flat-sequence {
          frame #0 {
            n199 = flat-sequence {
              frame #0 {
                w349 = "_" ("string")
                n200 = Get Date/Time In Seconds() -> (seconds since 1Jan1904=w346:timestamp)
                n201 = local read "RUN identifier"() -> (w353:string)
                n202 = call "LV_UNIXTIME.vi"("current time"=w346) -> ("date/time string"=w350:string)  [unwired: 9 in, 1 out]
                n203 = local read "Base Path"() -> (w354:path)
                n204 = Concatenate Strings(w353, w349, w350, w349, "FIle suffix 1", ".bmp" ("string")) -> (w359:string)
                n205 = control-ref of="Graph 1"() -> (w351:refnum<vi>)
                n206 = Build Path(base path=w354, name or relative path=w359) -> (appended path=w358:path)
                n207 = invoke on="Invoke Node" class="XYGraph (strict)" method="Export Image"(reference=w351, "FileType"=enum32{"BMP", "EPS", "EMF", "PICT"}."BMP" ("File Type"), "Target"=enum32{"File", "Clipboard"}."File", "Path"=w358, "HideGrid"=FALSE ("Hide Grid"), "Overwrite"=TRUE ("Always Overwrite")) -> ()  [unwired: 2 in, 8 out]
              }
              frame #1 {
                n208 = local write "Take Screenshot! 1"(FALSE ("Take Screenshot! 1")) -> ()
              }
            }
          }
        }
      }
      event "Take Screenshot! 2": Value Change {
        n209 = event-data() -> ()  [unwired: 1 in, 6 out]
        n210 = flat-sequence {
          frame #0 {
            n211 = flat-sequence {
              frame #0 {
                w365 = "_" ("string")
                n212 = Get Date/Time In Seconds() -> (seconds since 1Jan1904=w361:timestamp)
                n213 = local read "RUN identifier"() -> (w368:string)
                n214 = call "LV_UNIXTIME.vi"("current time"=w361) -> ("date/time string"=w366:string)  [unwired: 9 in, 1 out]
                n215 = local read "Base Path"() -> (w369:path)
                n216 = Concatenate Strings(w368, w365, w366, w365, "FIle suffix 2", ".bmp" ("string")) -> (w374:string)
                n217 = control-ref of="Graph 2"() -> (w362:refnum<vi>)
                n218 = Build Path(base path=w369, name or relative path=w374) -> (appended path=w373:path)
                n219 = invoke on="Invoke Node" class="XYGraph (strict)" method="Export Image"(reference=w362, "FileType"=enum32{"BMP", "EPS", "EMF", "PICT"}."BMP" ("File Type"), "Target"=enum32{"File", "Clipboard"}."File", "Path"=w373, "HideGrid"=FALSE ("Hide Grid"), "Overwrite"=TRUE ("Always Overwrite")) -> ()  [unwired: 2 in, 8 out]
              }
              frame #1 {
                n220 = local write "Take Screenshot! 2"(FALSE ("Take Screenshot! 1")) -> ()
              }
            }
          }
        }
      }
      event "Take Screenshot! 3": Value Change {
        n221 = event-data() -> ()  [unwired: 1 in, 6 out]
        n222 = flat-sequence {
          frame #0 {
            n223 = flat-sequence {
              frame #0 {
                w380 = "_" ("string")
                n224 = Get Date/Time In Seconds() -> (seconds since 1Jan1904=w378:timestamp)
                n225 = local read "RUN identifier"() -> (w383:string)
                n226 = call "LV_UNIXTIME.vi"("current time"=w378) -> ("date/time string"=w381:string)  [unwired: 9 in, 1 out]
                n227 = local read "Base Path"() -> (w384:path)
                n228 = Concatenate Strings(w383, w380, w381, w380, "FIle suffix 3", ".bmp" ("string")) -> (w389:string)
                n229 = control-ref of="Graph 3"() -> (w376:refnum<vi>)
                n230 = Build Path(base path=w384, name or relative path=w389) -> (appended path=w388:path)
                n231 = invoke on="Invoke Node" class="XYGraph (strict)" method="Export Image"(reference=w376, "FileType"=enum32{"BMP", "EPS", "EMF", "PICT"}."BMP" ("File Type"), "Target"=enum32{"File", "Clipboard"}."File", "Path"=w388, "HideGrid"=FALSE ("Hide Grid"), "Overwrite"=TRUE ("Always Overwrite")) -> ()  [unwired: 2 in, 8 out]
              }
              frame #1 {
                n232 = local write "Take Screenshot! 3"(FALSE ("Take Screenshot! 1")) -> ()
              }
            }
          }
        }
      }
      event "Take Screenshot! 4": Value Change {
        n233 = event-data() -> ()  [unwired: 1 in, 6 out]
        n234 = flat-sequence {
          frame #0 {
            n235 = flat-sequence {
              frame #0 {
                w395 = "_" ("string")
                n236 = Get Date/Time In Seconds() -> (seconds since 1Jan1904=w393:timestamp)
                n237 = local read "RUN identifier"() -> (w398:string)
                n238 = call "LV_UNIXTIME.vi"("current time"=w393) -> ("date/time string"=w396:string)  [unwired: 9 in, 1 out]
                n239 = local read "Base Path"() -> (w399:path)
                n240 = Concatenate Strings(w398, w395, w396, w395, "FIle suffix 4", ".bmp" ("string")) -> (w404:string)
                n241 = control-ref of="Graph 4"() -> (w391:refnum<vi>)
                n242 = Build Path(base path=w399, name or relative path=w404) -> (appended path=w403:path)
                n243 = invoke on="Invoke Node" class="XYGraph (strict)" method="Export Image"(reference=w391, "FileType"=enum32{"BMP", "EPS", "EMF", "PICT"}."BMP" ("File Type"), "Target"=enum32{"File", "Clipboard"}."File", "Path"=w403, "HideGrid"=FALSE ("Hide Grid"), "Overwrite"=TRUE ("Always Overwrite")) -> ()  [unwired: 2 in, 8 out]
              }
              frame #1 {
                n244 = local write "Take Screenshot! 4"(FALSE ("Take Screenshot! 1")) -> ()
              }
            }
          }
        }
      }
      event "Stop Button": Value Change {
        n245 = event-data() -> ()  [unwired: 1 in, 6 out]
      }
    }
    n246 = local write "Take Screenshot! 4"(FALSE ("Take Screenshot! 1")) -> ()
    n247 = local write "Take Screenshot! 1"(FALSE ("Take Screenshot! 1")) -> ()
    n248 = local write "Take Screenshot! 2"(FALSE ("Take Screenshot! 1")) -> ()
    n249 = local write "Take Screenshot! 3"(FALSE ("Take Screenshot! 1")) -> ()
    n250 = Wait (ms)(milliseconds to wait=u32 1000) -> ()  [unwired: 1 out]
  }
  n251 = while {
    shift-right: [w477] -> w24
    shift-left: refnum<class "USBData.lvclass"> refnum ("USBData.lvclass") -> [w481]
    shift-right: [w473] -> w23
    shift-left: errorcluster {"status"=FALSE, "code"=0, "source"=""} ("error in (no error)") -> [w480]
    tunnel: "RUN identifier" -> [w410]
    tunnel: "Base Path" -> [w409]
    shift-right: [w453] -> w17
    shift-left: errorcluster {"status"=FALSE, "code"=0, "source"=""} ("error in (no error)") -> [w471]
    shift-right: [w454] -> w18
    shift-left: refnum<class "LSI218Data.lvclass"> refnum ("LSI218Data.lvclass") -> [w470]
    shift-right: [w439] -> w14
    shift-left: refnum<class "LSI336Data.lvclass"> refnum ("LSI336Data.lvclass") -> [w450]
    shift-right: [w438] -> w13
    shift-left: w3 -> [w449]
    shift-right: [w426] -> _
    shift-left: errorcluster {"status"=FALSE, "code"=0, "source"=""} ("error in") -> [w427]
    shift-right: [w415] -> w7
    shift-left: refnum<class "USBData.lvclass"> refnum ("USBData.lvclass") -> [w424]
    shift-right: [w414] -> w6
    shift-left: errorcluster {"status"=FALSE, "code"=0, "source"=""} ("error in (no error)") -> [w423]
    shift-right: [w408] -> _
    shift-left: w3 -> [w407]
    i -> [w422]
    stop <- "Stop Button" stop-if-true
    w434 = u32 24 ("Number of Rows")
    w446 = T14 [] ("appended array")
    w464 = T14 [] ("appended array")
    n252 = control-ref of="Plot selecter LSI218(2)\n    1      2     3     4"() -> (w432:refnum<vi>)
    n253 = control-ref of="Plot selecter LSI218(1)\n    1      2     3     4"() -> (w433:refnum<vi>)
    n254 = control-ref of="Plot selecter LSI336 \n     1      2     3     4"() -> (w431:refnum<vi>)
    n255 = Equal?(x=w422, y=0) -> (x = y?=w411:bool)
    n256 = property on="Property Node" class="Arr (strict)"(reference=w433, "Number of Rows"=w434) -> ()  [unwired: 1 in, 2 out]
    n257 = property on="Property Node" class="Arr (strict)"(reference=w432, "Number of Rows"=w434) -> ()  [unwired: 1 in, 2 out]
    n258 = case shown="False" w411 {
      tunnel: w481 -> [w1121 w1145]
      tunnel: w480 -> [w1115 w1143]
      tunnel: w422 -> [w1106 _]
      tunnel: [w1113 w1140] -> w473
      tunnel: [w1110 w1139] -> w425
      tunnel: [w1111 w1138] -> w477
      tunnel: [w1101 w1133] -> w478
      tunnel: w410 -> [_ w1131]
      tunnel: w409 -> [_ w1130]
      tunnel: [w1100 w1127] -> w428
      frame False {
        n259 = call-dynamic "USBData_measure.vi"("USBData in"=w1121, "DAQ sample #"=i64 5, "DAQ timeout"=100.0 ("DAQ timeout (def: 100)"), "MeasurementIndex"=w1106, "error in (no error)"=w1115, "save every ... measurements"="Record interval") -> ("USBData out"=w1120:refnum<class "USBData.lvclass">, "TimeMeasuremeent"=w1117:timestamp, "Status"=→"USB6210 Status":T5, "LastDataAcquired"=w1102:dbl[], "error out"=w1116:errorcluster)  [unwired: 3 in, 2 out]
        "Time of Last Measurement (USB6210)" <- w1117
        "Last Vol\n(USB6210)" <- w1102
        n260 = call-dynamic "USBData_convert.vi"("Save every ... measurements"="Record interval", "MeasurementIndex"=w1106, "error in (no error)"=w1116, "LastDataAcquired"=w1102, "TimeMeasuremeent"=w1117, "USBData in"=w1120) -> ("error out"=w1114:errorcluster, "LeakDet_FULL"=w1109:dbl, "LastDataConverted"=w1103:dbl[], "USBData out"=w1112:refnum<class "USBData.lvclass">)  [unwired: 2 in]
        n261 = call "USBData_read.vi"("USBData in"=w1112, "error in (no error)"=w1114) -> ("Status"=w1104:T5, "USBData out"=w1111:refnum<class "USBData.lvclass">, "Data"=w1110:T15, "Basic"=w1101:T16, "error out"=w1113:errorcluster)  [unwired: 2 in, 2 out]
        n262 = local write "USB6210 Status"(w1104) -> ()
        n263 = Unbundle By Name(w1101) -> ("ReadLeakDet?"=w1108:bool)
        n264 = Unbundle By Name(w1101) -> ("Labels"=w1100:string[])
        n265 = case shown="False" w1108 {
          tunnel: w1103 -> [w1122 w1125]
          tunnel: w1109 -> [_ w1124]
          tunnel: [w1122 w1123] -> w1107
          frame False {
          }
          frame True {
            n266 = Build Array (concatenate)(w1125, w1124) -> (w1123:dbl[])
          }
        }
        "Last Data \n(USB6210)" <- w1107
      }
      frame True {
        n267 = Get Date/Time In Seconds() -> (seconds since 1Jan1904=w1132:timestamp)
        n268 = call-dynamic "USBData_initialize.vi"("USBData in"=w1145, "SeriesSetting"="USB6210 Config", "BasePath"=w1130, "RunName"=w1131, "FileName"="InstName (USB6210)", "error in (no error)"=w1143, "RUN start time"=w1132) -> ("Status"=w1126:T5, "USBData out"=w1141:refnum<class "USBData.lvclass">, "error out"=w1142:errorcluster)  [unwired: 4 in, 2 out]
        n269 = local write "USB6210 Status"(w1126) -> ()
        n270 = call "USBData_read.vi"("USBData in"=w1141, "error in (no error)"=w1142) -> ("Status"=w1129:T5, "USBData out"=w1138:refnum<class "USBData.lvclass">, "Data"=w1139:T15, "Basic"=w1133:T16, "error out"=w1140:errorcluster)  [unwired: 2 in, 2 out]
        n271 = local write "USB6210 Status"(w1129) -> ()
        n272 = Unbundle By Name(w1133) -> ("ReadLeakDet?"=w1137:bool, "Labels"=w1127:string[])
        n273 = Array Size(array=w1127) -> (size(s)=w1136:i32)
        n274 = case shown="True" w1137 {
          tunnel: w1136 -> [w1146 w1148]
          tunnel: [w1146 w1147] -> w1134
          frame False {
          }
          frame True {
            n275 = Add(x=w1148, y=1) -> (x+y=w1147:i32)
          }
        }
        n276 = Initialize Array(TRUE ("Activate 2"), w1134) -> ()  [unwired: 1 out]
      }
    }
    "error out (USB6210)" <- w473
    n277 = case shown="False" w411 {
      tunnel: [w974 w986] -> w438
      tunnel: [w964 w985] -> w448
      tunnel: [w973 w984] -> w439
      tunnel: [w972 timestamp[] [] ("TimeArray")] -> w444
      tunnel: [w971 dbl[][] [] ("DataArray")] -> w445
      tunnel: w450 -> [w970 w981]
      tunnel: w449 -> [w969 w980]
      tunnel: w410 -> [_ w978]
      tunnel: w422 -> [w965 _]
      tunnel: w409 -> [_ w975]
      frame False {
        n278 = local read "Record interval"() -> (w962:i64)
        n279 = call-dynamic "LSI336Data_measure.vi"("LSI336Data in"=w970, "MeasurementIndex"=w965, "error in (no error)"=w969, "save every ... measurements"=w962) -> ("Active?"=→"Active?\n(LSI336)":bool[], "TimeMeasuremeent"=→"Time of Last Measurement (LSI336) 2":timestamp, "LSI336Data out"=w973:refnum<class "LSI336Data.lvclass">, "LastData"=→"Last Data \nLSI336":dbl[], "LastMeasurementConfig"=→"LastMeasurementConfig (336)":T11, "DataArray"=w971:dbl[][], "Status"=w964:u16, "TimeArray"=w972:timestamp[], "error out"=w974:errorcluster)  [unwired: 3 in]
      }
      frame True {
        n280 = Get Date/Time In Seconds() -> (seconds since 1Jan1904=w987:timestamp)
        n281 = call-dynamic "LSI336Data_initialize.vi"("LSI336Data in"=w981, "RunName"=w978, "InstName"="InstName (LSI336)", "FileFormat"="FileFormat (336)", "LSI336Settings(X, Y)"="LSI336Settings(X,Y)", "RUN start time"=w987, "error in (no error)"=w980, "base path"=w975) -> ("LSI336Data out"=w984:refnum<class "LSI336Data.lvclass">, "Status"=w985:T6, "AllLabels"=→"Labels LSI336":string[], "error out"=w986:errorcluster)  [unwired: 4 in]
      }
    }
    "LSI336 Status" <- w448
    "error out (LSI336)" <- w438
    n282 = case shown="False" w411 {
      tunnel: [w695 w723] -> w414
      tunnel: [w692 w722] -> w421
      tunnel: [w693 w721] -> w415
      tunnel: [w684 w716] -> w420
      tunnel: [w683 w713] -> _
      tunnel: w424 -> [w682 w711]
      tunnel: w409 -> [_ w710]
      tunnel: w410 -> [_ w709]
      tunnel: w423 -> [w681 w708]
      tunnel: w422 -> [w680 _]
      frame False {
        n283 = local read "Record interval"() -> (w679:i64)
        n284 = call-dynamic "USBData_measure.vi"("USBData in"=w682, "DAQ sample #"=i64 5, "DAQ timeout"=100.0 ("DAQ timeout (def: 100)"), "MeasurementIndex"=w680, "error in (no error)"=w681) -> ("USBData out"=w701:refnum<class "USBData.lvclass">, "TimeMeasuremeent"=w698:timestamp, "Status"=→"USB6218 Status":T5, "LastDataAcquired"=w685:dbl[], "error out"=w697:errorcluster)  [unwired: 4 in, 2 out]